vi "UHR-Fleezers Control (host) - 10.3.vi"() -> ()   [LabVIEW 2010] (continued)
        n744 = property on="Mean" class="DigNum (strict)"("Caption.Text"=w1860) -> ()  [unwired: 2 in, 2 out]
        n745 = property on="Difference" class="DigNum (strict)"("Caption.Text"=w1859) -> ()  [unwired: 2 in, 2 out]
      }
    }
    n746 = local read "Tether"() -> (w1089:bool)
    n747 = Absolute Value(x=w1062) -> (abs(x)=w1059:dbl)
    n748 = Absolute Value(x=w1061) -> (abs(x)=w1058:dbl)
    n749 = Add(x=w1059, y=w1058) -> (x+y=w1137:dbl)
    n750 = Subtract(x=w1059, y=w1058) -> (x-y=→"Difference":dbl)
    n751 = feedback #18(w1080) -> (w1079:dbl[])
    n752 = Divide(x=w1137, y=2.0) -> (x/y=w1088:dbl)
    "Mean" <- w1088
    n753 = case shown="True" w1089 {
      tunnel: w1088 -> [_ w1404]
      frame False {
      }
      frame True {
        n754 = Greater?(x="Lost Tether Alarm Threshold (pN)", y=w1404) -> (0:w1402:bool)
        n755 = case shown="True" w1402 {
          frame False {
          }
          frame True {
            n756 = flat-sequence {
              frame #0 {
                # "stop only if saving"
                n757 = local read "Saving..."() -> (w1417:bool)
                n758 = And(x=w1417, y="TA Cancel Save?") -> (x .and. y?=w1416:bool)
                n759 = local write "Stop Saving"(w1416) -> ()
              }
              frame #1 {
                n760 = case shown="True" "TA Green Off?" {
                  frame False {
                  }
                  frame True {
                    w1420 = FALSE ("Fl. Triggered...")
                    n761 = local write "Fl. Triggered..."(w1420) -> ()
                    n762 = property on="Green Laser ON/Interlacing" class="Bool (strict)"("Val(Sgnl)"=w1420) -> ()  [unwired: 2 in, 2 out]
                  }
                }
              }
            }
            n763 = local read "Time tether formed"() -> (w1411:timestamp)
            n764 = Get Date/Time In Seconds() -> (seconds since 1Jan1904=w1412:timestamp)
            n765 = Subtract(x=w1412, y=w1411) -> (x-y=w1410:dbl)
            n766 = Number To Decimal String(number=w1410) -> (decimal integer string=w1407:string)  [unwired: 1 out]
            n767 = local read "Messages"() -> (w1414:string)
            n768 = call <vilib>:"Beep.vi"() -> ()  [unwired: 3 in, 9 out]
            n769 = Concatenate Strings("Lost tether (" ("Message to add"), w1407, " s)." ("string")) -> (w1409:string)
            n770 = local write "Tether"(FALSE ("Tether")) -> ()
            n771 = call "Update messages.vi"("Message to add"=w1409, "Old message string"=w1414) -> ("New message string"=w1413:string)
            n772 = local write "Messages"(w1413) -> ()
            n773 = property on="Trap Pos. FB ON" class="Bool (strict)"("Val(Sgnl)"=FALSE ("Value (Signaling)")) -> ()  [unwired: 2 in, 2 out]
          }
        }
      }
    }
    n774 = Build Array (concatenate)(w1080, w1079) -> (w1078:dbl[])
    n775 = Split 1D Array(array=w1078, index=w957) -> (first subarray=w1074:dbl[])  [unwired: 1 out]
    n776 = feedback-in #18(w1074) -> ()
    n777 = call <vilib>:"Mean.vi"("X"=w1074) -> ("mean"=w1073:dbl)  [unwired: 1 out]
    "Bead Mean (nm)" <- w1073
    n778 = Subtract(x=w1074, y=w1073) -> (x-y=w1072:dbl[])
    n779 = Square(x=w1072) -> (x^2=w1071:dbl[])
    n780 = call <vilib>:"Mean.vi"("X"=w1071) -> ("mean"=w1070:dbl)  [unwired: 1 out]
    n781 = Square Root(x=w1070) -> (sqrt(x)=w1069:dbl)
    n782 = Multiply(x=10.0, y=w1069) -> (x*y=→"RMS (Ang)":dbl)
    n783 = xnode "Read/Write Control"("FPGA VI Reference In"=w1113, "error in"=w1112) -> ("FPGA VI Reference Out"=w1231:T19, "error out"=w1225:errorcluster, "AI2 Y Sum Set 1"=w1221:i16, "AI2 Y Sum Set 2"=w1220:i16, "AI1 X Set 1"=w992:fxp<+/-,16,1>, "AI1 X Set 2"=w991:fxp<+/-,16,1>, "Trap Pos FB Int Signal"=→"Trap Pos FB Int Signal":fxp<+/-,24,9>, "Trap Pos FB Int-Norm Signal"=→"Trap Pos FB Int-Norm Signal":fxp<+/-,16,1>, "Trap Pos FB Action"=w985:i64, "Scanning"=→"AOD Scanning":bool, "Scan I"=→"AOD Scan I":u64, "Scanning MCL"=w1223:bool, "Scan I (MCL)"=→"MCL Scan I":u64, "Green FB Signals"=w1160:T32)  [unwired: 1 out]
    "MCL Scanning" <- w1223
    "Trap Pos FB Action" <- w985
    n784 = local read "AI2 (V)"() -> (w1222:cluster{"Set 1":dbl, "Set 2":dbl})
    n785 = Bundle By Name(cluster=w1222, "Set 1"=w1221, "Set 2"=w1220) -> (w1218:cluster{"Set 1":dbl, "Set 2":dbl})
    n786 = Divide(x=w985, y=327.67) -> (x/y=→"Action (%)":dbl)
    n787 = local read "Trap X (AI1)"() -> (w1005:T10)
    n788 = Divide(x=w1218, y=3276.7) -> (x/y=w1217:cluster{"Set 1":dbl, "Set 2":dbl})
    n789 = local write "AI2 (V)"(w1217) -> ()
    n790 = Bundle(cluster=w1005, "Trap 1"=w992, "Trap 2"=w991) -> (→"Trap X (AI1)":T10)
    n791 = Divide(x=w1160, y=3276.7) -> (x/y=w1156:T41)
    n792 = Unbundle By Name(w1156) -> ("Green FB Ch 0"=w1159:dbl, "Green FB Ch 1"=w1158:dbl, "Green FB Ch 2"=w1157:dbl)
    n793 = Divide(x=w1159, y=w1157) -> (x/y=w1155:dbl)
    n794 = Divide(x=w1158, y=w1157) -> (x/y=w1154:dbl)
    n795 = flat-sequence "To save data" {
      tunnel: [w3725] -> w1243
      tunnel: [w3726] -> w1242
      tunnel: w1191 -> [w3719]
      tunnel: w1076 -> [w3723]
      tunnel: ["Save Calibration"] -> w1214
      tunnel: w1211 -> [w3722]
      tunnel: [w3715] -> w1210
      tunnel: [w3712] -> w1209
      tunnel: [w3709] -> w1208
      tunnel: w1190 -> [w3711]
      tunnel: w1095 -> [w3705]
      tunnel: [w3705] -> w1094
      tunnel: ["Start Saving"] -> w1050
      tunnel: [w3699] -> w973
      tunnel: [w3698] -> w972
      tunnel: w1243 -> [w3960]
      tunnel: w1242 -> [w3959]
      tunnel: w974 -> [w3958]
      tunnel: w1214 -> [w3957]
      tunnel: w1210 -> [w3955]
      tunnel: w1209 -> [w3954]
      tunnel: w1208 -> [w3953]
      tunnel: w1063 -> [w3952]
      tunnel: w1105 -> [w3951]
      tunnel: w1094 -> [w3950]
      tunnel: w1050 -> [w3949]
      tunnel: w1048 -> [w3948]
      tunnel: w1024 -> [w3947]
      tunnel: w973 -> [w3946]
      tunnel: w972 -> [w3945]
      tunnel: w971 -> [w3944]
      frame #0 {
        n796 = Or(x="Save N Sets", y="Start Saving") -> (x .or. y?=w3706:bool)
        n797 = To Double Precision Float(number=w3722) -> (double precision float=w3716:dbl)
        n798 = Build Array(w3706, "Save Calibration", w3719, w3711) -> (w3721:bool[])
        n799 = Compound Arithmetic op=OR("Save Calibration", w3719, w3706, w3711) -> (w3724:bool)
        n800 = Boolean Array To Number(Boolean array=w3721) -> (number=w3718:u32)
        n801 = feedback #19(FALSE ("Save APD Data\nwith Trap Data")) -> (w3700:bool)
        n802 = feedback #20(refnum<k0> refnum) -> (w3727:refnum<file>)
        n803 = feedback #21(refnum<k0> refnum) -> (w3702:refnum<file>)
        n804 = feedback #22(FALSE ("Save APD Data\nwith Trap Data")) -> (w3710:bool)
        n805 = feedback #23(refnum<k0> refnum) -> (w3713:refnum<file>)
        n806 = feedback #24(0) -> (w3729:i32)
        n807 = feedback #25() -> (w3717:u32)  [unwired: 1 out]
        n808 = case shown="True" w3724 {
          tunnel: [w3736 1] -> w3725
          tunnel: w3729 -> [w3738 _]
          tunnel: [w3737 w3756] -> w3726
          tunnel: w3727 -> [w3737 _]
          tunnel: w3723 -> [_ w3776]
          tunnel: w3716 -> [_ w3774]
          tunnel: w3718 -> [_ w3777]
          tunnel: [w3735 w3755] -> w3715
          tunnel: w3717 -> [w3735 _]
          tunnel: [w3734 w3753] -> w3712
          tunnel: w3713 -> [w3734 _]
          tunnel: [w3733 w3752] -> w3709
          tunnel: w3710 -> [w3733 _]
          tunnel: "Start Saving" -> [_ w3750]
          tunnel: w3705 -> [_ w3749]
          tunnel: [w3732 w3740] -> w3698
          tunnel: w3702 -> [w3732 _]
          tunnel: [w3731 w3739] -> w3699
          tunnel: w3700 -> [w3731 _]
          frame False {
            n809 = Increment(x=w3738) -> (x+1=w3736:i32)
          }
          frame True {
            w3746 = FALSE ("Start Saving")
            w3751 = 9.0  # File Version
            w3759 = FALSE ("prepend array or string size? (T)")
            w3757 = T34."big-endian, network order" ("byte order (0:big-endian, network order)")
            n810 = local read "BD 1 Frequency 1 (MHz)"() -> (w3773:dbl)
            n811 = local read "BD 2 Frequency 1 (MHz)"() -> (w3772:dbl)
            n812 = local read "BD 1 Frequency 2 (MHz)"() -> (w3771:dbl)
            n813 = local read "BD 2 Frequency 2 (MHz)"() -> (w3770:dbl)
            n814 = local read "BD 1 Frequency 3 (MHz)"() -> (w3769:dbl)
            n815 = local read "BD 2 Frequency 3 (MHz)"() -> (w3768:dbl)
            n816 = Array Size(array=w3749) -> (size(s)=w3748:i32)
            n817 = To Double Precision Float(number=w3748) -> (double precision float=w3747:dbl)
            n818 = local write "Save Calibration"(w3746) -> ()
            n819 = local write "Start Saving"(w3746) -> ()
            n820 = Build Array("Save APD Data\nwith Trap Data", "Save Trap Pos. Data") -> (w3743:bool[])
            n821 = Boolean Array To Number(Boolean array=w3743) -> (number=w3742:u32)
            n822 = Build Array(w3773, w3772, w3771, w3770, w3769, w3768) -> (w3767:dbl[])
            n823 = case shown="4" w3777 {
              tunnel: w3776 -> [w3848 w3868 w3884 w3922]
              tunnel: w3747 -> [w3853 w3875 w3904 w3941]
              tunnel: w3774 -> [w3852 w3874 w3903 w3940]
              tunnel: [w3849 w3870 w3895 w3932] -> w3765
              tunnel: [w3840 "Cal sets to save" w3885 w3923] -> w3755
              tunnel: w3767 -> [w3850 w3871 w3897 w3934]
              tunnel: "Save APD Data\nwith Trap Data" -> [w3847 _ w3881 w3920]
              tunnel: [w3847 w3862 w3881 w3920] -> w3752
              tunnel: w3751 -> [w3843 w3863 w3879 w3918]
              tunnel: w3750 -> [w3842 _ _ _]
              tunnel: [w3833 w3862 w3878 w3908] -> w3739
              tunnel: "Save Trap Pos. Data" -> [w3833 _ w3878 w3908]
              tunnel: w3742 -> [w3832 _ w3877 w3907]
              frame 1, Default {
                # "timeseries"
                n824 = case shown="True" "Profile" {
                  tunnel: [w3856 w3860] -> w3837
                  tunnel: [w3856 w3859] -> w3836
                  tunnel: [w3856 w3858] -> w3835
                  tunnel: [w3856 w3857] -> w3834
                  frame False {
                    w3856 = 0.0 ("f")
                  }
                  frame True {
                    n825 = local read "Current Position"() -> (w3861:cluster{dbl, dbl, dbl})
                    n826 = local read "Y change (mm)"() -> (w3857:dbl)
                    n827 = Unbundle(w3861) -> (w3860:dbl, w3859:dbl, w3858:dbl)
                  }
                }
                n828 = local read "Save ave N"() -> (w3855:dbl)
                n829 = Multiply(x=w3855, y=w3848) -> (x*y=w3854:dbl)
                n830 = To Double Precision Float(number=w3832) -> (double precision float=w3846:dbl)
                n831 = Build Array(w3843, w3848, w3854, w3853, w3852, 0.0 ("f")) -> (w3851:dbl[])
                n832 = Build Array(w3846, w3837, w3836, w3835, w3834) -> (w3844:dbl[])
                n833 = Select(t=u32 4000000000, s=w3842, f="N sets to save") -> (s? t:f=w3840:u32)
                n834 = Build Array (concatenate)(w3851, w3850, w3844) -> (w3849:dbl[])
              }
              frame 2 {
                w3865 = 0.0 ("f")
                w3862 = FALSE ("Save APD Data\nwith Trap Data")
                # "calibration"
                n835 = Boolean To (0,1)(Boolean=w3862) -> (0, 1=w3867:i16)
                n836 = To Double Precision Float(number=w3867) -> (double precision float=w3866:dbl)
                n837 = Build Array(w3866, w3865, w3865, w3865, w3865) -> (w3864:dbl[])
                n838 = Build Array(w3863, w3868, w3868, w3875, w3874, 1.0 ("t")) -> (w3872:dbl[])
                n839 = Build Array (concatenate)(w3872, w3871, w3864) -> (w3870:dbl[])
                "Calibrating Trap..." <- TRUE ("Calibrating...")
              }
              frame 4 {
                w3882 = 0.0 ("f")
                # "scan dir (x/y = 0/1)"
                # "cycles/step"
                # "n scans (f/b)"
                # "steps"
                # "freq. range"
                # "AOD raster scan"
                n840 = local read "Number of F/B Scans (AOD)"() -> (w3889:u16)
                n841 = local read "Cycles/step (AOD)"() -> (w3891:u64)
                n842 = local read "Scan Range (MHz)"() -> (w3894:dbl)
                n843 = local read "Scan steps (AOD)"() -> (w3893:u64)
                n844 = local read "Scan BD"() -> (w3901:bool)
                n845 = local read "Save ave N"() -> (w3906:dbl)
                n846 = Boolean To (0,1)(Boolean=w3901) -> (0, 1=w3900:i16)
                n847 = To Double Precision Float(number=w3889) -> (double precision float=w3888:dbl)
                n848 = To Double Precision Float(number=w3893) -> (double precision float=w3892:dbl)
                n849 = To Double Precision Float(number=w3891) -> (double precision float=w3890:dbl)
                n850 = To Double Precision Float(number=w3900) -> (double precision float=w3899:dbl)
                n851 = Multiply(x=w3906, y=w3884) -> (x*y=w3905:dbl)
                n852 = To Double Precision Float(number=w3877) -> (double precision float=w3883:dbl)
                n853 = Build Array(w3883, w3882, w3882, w3882, w3882) -> (w3880:dbl[])
                n854 = local read "N sets should be saved"() -> (w3886:dbl)
                n855 = Build Array(w3899, w3894, w3892, w3890, w3888) -> (w3896:dbl[])
                n856 = Build Array(w3879, w3884, w3905, w3904, w3903, 2.0 ("t")) -> (w3898:dbl[])
                n857 = Round Toward +Infinity(x=w3886) -> (ceil(x): smallest int >= x=w3887:dbl)
                n858 = Build Array (concatenate)(w3898, w3897, w3880, w3896) -> (w3895:dbl[])
                n859 = To Unsigned Long Integer(number=w3887) -> (unsigned 32bit integer=w3885:u32)
              }
              frame 8 {
                w3915 = 0.0 ("f")
                # "MCL raster scan"
                n860 = local read "Number of scans (MCL)"() -> (w3910:u64)
                n861 = local read "Scan lines (y)"() -> (w3909:u64)
                n862 = local read "2D or 1D Scan"() -> (w3912:bool)
                n863 = local read "Scan Range (V)\n(of steps)"() -> (w3931:dbl)
                n864 = local read "Fast Scan Dir"() -> (w3938:bool)
                n865 = local read "Cycles/step (MCL)"() -> (w3928:u64)
                n866 = local read "Scan steps (MCL)"() -> (w3930:u64)
                n867 = Select(t=w3909, s=w3912, f=w3910) -> (s? t:f=w3911:u64)
                n868 = Boolean To (0,1)(Boolean=w3912) -> (0, 1=w3914:i16)
                n869 = local read "Save ave N"() -> (w3943:dbl)
                n870 = local read "Initial X"() -> (w3917:dbl)
                n871 = local read "Initial Y"() -> (w3916:dbl)
                n872 = To Double Precision Float(number=w3914) -> (double precision float=w3913:dbl)
                n873 = Boolean To (0,1)(Boolean=w3938) -> (0, 1=w3937:i16)
                n874 = To Double Precision Float(number=w3911) -> (double precision float=w3926:dbl)
                n875 = To Double Precision Float(number=w3930) -> (double precision float=w3929:dbl)
                n876 = To Double Precision Float(number=w3928) -> (double precision float=w3927:dbl)
                n877 = To Double Precision Float(number=w3937) -> (double precision float=w3936:dbl)
                n878 = Multiply(x=w3943, y=w3922) -> (x*y=w3942:dbl)
                n879 = To Double Precision Float(number=w3907) -> (double precision float=w3921:dbl)
                n880 = local read "N sets should be saved (MCL)"() -> (w3924:dbl)
                n881 = Build Array(w3921, w3913, w3915, w3915, w3915) -> (w3919:dbl[])
                n882 = Build Array(w3936, w3931, w3929, w3927, w3926, w3917, w3916) -> (w3933:dbl[])
                n883 = Build Array(w3918, w3922, w3942, w3941, w3940, 3.0 ("t")) -> (w3935:dbl[])
                n884 = Round Toward +Infinity(x=w3924) -> (ceil(x): smallest int >= x=w3925:dbl)
                n885 = Build Array (concatenate)(w3935, w3934, w3919, w3933) -> (w3932:dbl[])
                n886 = To Unsigned Long Integer(number=w3925) -> (unsigned 32bit integer=w3923:u32)
              }
            }
            n887 = local read "Index"() -> (w3782:dbl)
            n888 = call "Create new save file.vi"("Insert"="", "Ext"=".dat", "Index In"=w3782) -> ("Path Out"=w3741:path, "Index Out"=w3754:dbl)
            n889 = local write "Save file name"(w3741) -> ()
            n890 = local write "Index"(w3754) -> ()
            n891 = local write "Save index"(w3754) -> ()
            n892 = Array Size(array=w3765) -> (size(s)=w3766:i32)
            n893 = Open/Create/Replace File(file path (use dialog)=w3741, operation (0:open)=T33."create", access (0:read/write)=enum16{"read/write", "read-only", "write-only"}."write-only") -> (refnum out=w3779:refnum<file>)  [unwired: 1 in, 4 out]
            n894 = local write "Saving..."(TRUE ("Saving...")) -> ()
            n895 = To Double Precision Float(number=w3766) -> (double precision float=w3764:dbl)
            n896 = String Length(string="Comment (data description)") -> (length=w3762:i32)
            n897 = To Double Precision Float(number=w3762) -> (double precision float=w3761:dbl)
            n898 = Deny Access(7:w3779) -> (3:w3778:refnum<file>)  [unwired: 1 in, 2 out]
            n899 = Build Array (concatenate)(w3764, w3765, w3761) -> (w3763:dbl[])
            n900 = case "If fluorescence data to be saved" shown="True" w3752 {
              tunnel: w3741 -> [_ w3831]
              tunnel: [refnum<k0> refnum w3811] -> w3753
              frame False {
              }
              frame True {
                w3810 = 0.0
                n901 = local read "APD Integration Time (s)"() -> (w3816:dbl)
                n902 = local read "N APD Samp/step"() -> (w3809:dbl)
                n903 = Path To String(path=w3831) -> (string=w3830:string)
                n904 = String Length(string=w3830) -> (length=w3829:i32)
                n905 = Subtract(x=w3829, y=4) -> (x-y=w3827:i32)
                n906 = String Subset(string=w3830, length (rest)=w3827) -> (substring=w3826:string)  [unwired: 1 out]
                n907 = Build Array(w3816, w3809, w3810, w3810, w3810, w3810, w3810, w3810) -> (w3813:dbl[])
                n908 = Concatenate Strings(w3826, "_fl.dat" ("string")) -> (w3824:string)
                n909 = Array Size(array=w3813) -> (size(s)=w3815:i32)
                n910 = String To Path(string=w3824) -> (path=w3820:path)
                n911 = Open/Create/Replace File(file path (use dialog)=w3820, operation (0:open)=T33."create", access (0:read/write)=enum16{"read/write", "read-only", "write-only"}."write-only") -> (refnum out=w3821:refnum<file>)  [unwired: 1 in, 4 out]
                n912 = Deny Access(7:w3821) -> (3:w3817:refnum<file>)  [unwired: 1 in, 2 out]
                n913 = To Double Precision Float(number=w3815) -> (double precision float=w3814:dbl)
                n914 = Build Array (concatenate)(w3814, w3813) -> (w3812:dbl[])
                n915 = Write to Binary File(file (use dialog)=w3817, data=w3812, 5:FALSE ("prepend array or string size? (T)"), 9:T34."big-endian, network order" ("byte order (0:big-endian, network order)")) -> (refnum out=w3811:refnum<file>)  [unwired: 1 in, 3 out]
              }
            }
            n916 = case shown="True" w3739 {
              tunnel: w3741 -> [_ w3793]
              tunnel: [refnum<k0> refnum w3792] -> w3740
              frame False {
              }
              frame True {
                w3788 = 0.0 ("element")
                n917 = Path To String(path=w3793) -> (string=w3807:string)
                n918 = Build Array(w3788, w3788, w3788, w3788, w3788, w3788, w3788, w3788) -> (w3789:dbl[])
                n919 = String Length(string=w3807) -> (length=w3806:i32)
                n920 = Subtract(x=w3806, y=4) -> (x-y=w3804:i32)
                n921 = Array Size(array=w3789) -> (size(s)=w3791:i32)
                n922 = String Subset(string=w3807, length (rest)=w3804) -> (substring=w3803:string)  [unwired: 1 out]
                n923 = To Double Precision Float(number=w3791) -> (double precision float=w3790:dbl)
                n924 = Concatenate Strings(w3803, "_pos.dat" ("string")) -> (w3801:string)
                n925 = Build Array (concatenate)(w3790, w3789) -> (w3787:dbl[])
                n926 = String To Path(string=w3801) -> (path=w3797:path)
                n927 = Open/Create/Replace File(file path (use dialog)=w3797, operation (0:open)=T33."create", access (0:read/write)=enum16{"read/write", "read-only", "write-only"}."write-only") -> (refnum out=w3798:refnum<file>)  [unwired: 1 in, 4 out]
                n928 = Deny Access(7:w3798) -> (3:w3794:refnum<file>)  [unwired: 1 in, 2 out]
                n929 = Write to Binary File(file (use dialog)=w3794, data=w3787, 5:FALSE ("prepend array or string size? (T)"), 9:T34."big-endian, network order" ("byte order (0:big-endian, network order)")) -> (refnum out=w3792:refnum<file>)  [unwired: 1 in, 3 out]
              }
            }
            n930 = Write to Binary File(file (use dialog)=w3778, data=w3763, 5:w3759, 9:w3757) -> (refnum out=w3760:refnum<file>)  [unwired: 1 in, 3 out]
            n931 = Write to Binary File(file (use dialog)=w3760, data="Comment (data description)", 5:w3759, 9:w3757) -> (refnum out=w3756:refnum<file>)  [unwired: 1 in, 3 out]
          }
        }
        n932 = feedback-in #19(w3699) -> ()
        n933 = feedback-in #20(w3726) -> ()
        n934 = feedback-in #21(w3698) -> ()
        n935 = feedback-in #22(w3709) -> ()
        n936 = feedback-in #23(w3712) -> ()
        n937 = feedback-in #24(w3725) -> ()
        n938 = feedback-in #25(w3715) -> ()
      }
      frame #1 {
        n939 = local read "Saving..."() -> (w3956:bool)
        n940 = case shown="True" w3956 {
          tunnel: w3960 -> [_ w3970]
          tunnel: w3959 -> [_ w3984]
          tunnel: w3958 -> [_ w3980]
          tunnel: w3957 -> [_ w3979]
          tunnel: w3955 -> [_ w3978]
          tunnel: w3954 -> [_ w3973]
          tunnel: w3953 -> [_ w3972]
          tunnel: w3952 -> [_ w3971]
          tunnel: w3951 -> [_ w3969]
          tunnel: w3950 -> [_ w3967]
          tunnel: w3949 -> [_ w3966]
          tunnel: w3948 -> [_ w3965]
          tunnel: w3947 -> [_ w3964]
          tunnel: w3946 -> [_ w3963]
          tunnel: w3945 -> [_ w3962]
          tunnel: w3944 -> [_ w3961]
          frame False {
          }
          frame True {
            n941 = Multiply(x=w3970, y=w3969) -> (x*y=→"Time (s)":dbl)
            n942 = Less Or Equal?(x=w3970, y=w3978) -> (x <= y?=w3982:bool)
            n943 = Or(x="Stop Saving", y="Abort save 2") -> (x .or. y?=w3974:bool)
            n944 = Not(x=w3974) -> (.not. x?=w3983:bool)
            n945 = And(x=w3982, y=w3983) -> (x .and. y?=w3981:bool)
            n946 = case shown="True" w3981 {
              tunnel: w3984 -> [w3991 w4059]
              tunnel: [0.0 w4062] -> w3977
              tunnel: w3970 -> [_ w4060]
              tunnel: w3978 -> [_ w4061]
              tunnel: w3980 -> [_ w4056]
              tunnel: w3979 -> [_ _]
              tunnel: w3973 -> [w3989 w4049]
              tunnel: w3972 -> [w3988 w4050]
              tunnel: w3971 -> [_ w4048]
              tunnel: w3967 -> [_ w4047]
              tunnel: w3966 -> [_ w4001]
              tunnel: w3965 -> [_ w4040]
              tunnel: w3964 -> [_ w4018]
              tunnel: w3963 -> [w3985 w3999]
              tunnel: w3962 -> [w3986 w3998]
              tunnel: w3961 -> [_ w3995]
              frame False {
                w3987 = FALSE
                n947 = Close File(refnum=w3991) -> ()  [unwired: 1 in, 2 out]
                n948 = case shown="True" w3988 {
                  tunnel: w3989 -> [_ w3993]
                  frame False {
                  }
                  frame True {
                    n949 = Close File(refnum=w3993) -> ()  [unwired: 1 in, 2 out]
                  }
                }
                n950 = case shown="True" w3985 {
                  tunnel: w3986 -> [_ w3992]
                  frame False {
                  }
                  frame True {
                    n951 = Close File(refnum=w3992) -> ()  [unwired: 1 in, 2 out]
                  }
                }
                n952 = local write "Raster Scanning..."(w3987) -> ()
                n953 = local write "Calibrating Trap..."(w3987) -> ()
                n954 = call <vilib>:"Beep.vi"() -> ()  [unwired: 3 in, 9 out]
                n955 = local write "Stop Saving"(w3987) -> ()
                "Saving..." <- w3987
              }
              frame True {
                n956 = local read "Calibrating Trap..."() -> (w4051:bool)
                n957 = case "Write fl. data" shown="True" w4050 {
                  tunnel: w4049 -> [_ w4085]
                  tunnel: w4048 -> [_ w4084]
                  frame False {
                  }
                  frame True {
                    n958 = Write to Binary File(file (use dialog)=w4085, data=w4084, 5:FALSE ("prepend array or string size? (T)"), 9:T34."big-endian, network order" ("byte order (0:big-endian, network order)")) -> ()  [unwired: 1 in, 4 out]
                  }
                }
                n959 = Greater?(x="Save ave N", y=1.0) -> (0:w4054:bool)
                n960 = Not(x=w4051) -> (.not. x?=w4053:bool)
                n961 = And(x=w4053, y=w4054) -> (x .and. y?=w3996:bool)
                n962 = case shown="True" w3996 {
                  tunnel: w3995 -> [w4065 w4076]
                  tunnel: [w4065 w4068] -> w3994
                  tunnel: "Save ave N" -> [_ w4069]
                  frame False {
                  }
                  frame True {
                    w4066 = 2 ("dimension size")
                    n963 = Array Size(array=w4076) -> (size(s)=w4070:i32)
                    n964 = Divide(x=w4070, y=w4066) -> (x/y=w4074:dbl)
                    n965 = Reshape Array(w4076, w4074, w4066) -> (w4075:u64[][])
                    n966 = Transpose 2D Array(2D array=w4075) -> (transposed array=w4073:u64[][])
                    n967 = for {
                      tunnel: w4073 -> [w4078] mode=indexing
                      tunnel: [w4077] -> w4067 mode=indexing
                      tunnel: w4069 -> [w4079]
                      workers-P: _ -> [_]
                      n968 = call "downsample 1D array - U64.vi"("Ave N"=w4079, "Array In"=w4078) -> ("Array Out"=w4077:u64[])  [unwired: 1 in]
                    }
                    n969 = Transpose 2D Array(2D array=w4067) -> (transposed array=w4072:u64[][])
                    n970 = Divide(x=w4070, y=w4069) -> (x/y=w4071:dbl)
                    n971 = Reshape Array(w4072, w4071) -> (w4068:u64[])
                  }
                }
                n972 = case shown="True" w3996 {
                  tunnel: w4056 -> [w4088 w4100]
                  tunnel: [w4088 w4092] -> w4052
                  tunnel: "Save ave N" -> [_ w4093]
                  tunnel: w4047 -> [_ w4091]
                  frame False {
                  }
                  frame True {
                    n973 = Array Size(array=w4100) -> (size(s)=w4094:i32)
                    n974 = Array Size(array=w4091) -> (size(s)=w4090:i32)
                    n975 = Divide(x=w4094, y=w4090) -> (x/y=w4098:dbl)
                    n976 = Reshape Array(w4100, w4098, w4090) -> (w4099:i16[][])
                    n977 = Transpose 2D Array(2D array=w4099) -> (transposed array=w4097:i16[][])
                    n978 = for {
                      tunnel: w4097 -> [w4103] mode=indexing
                      tunnel: [w4102] -> w4089 mode=indexing
                      tunnel: w4093 -> [w4101]
                      workers-P: _ -> [_]
                      n979 = call "downsample 1D array - I16.vi"("Ave N"=w4101, "Array In"=w4103) -> ("Array Out"=w4102:i16[])  [unwired: 1 out]
                    }
                    n980 = Transpose 2D Array(2D array=w4089) -> (transposed array=w4096:i16[][])
                    n981 = Divide(x=w4094, y=w4093) -> (x/y=w4095:dbl)
                    n982 = Reshape Array(w4096, w4095) -> (w4092:i16[])
                  }
                }
                n983 = Index Array(array=w4018, index=1) -> (element=w4021:waveform(dbl))
                n984 = Index Array(array=w4018, index=0) -> (element=w4023:waveform(dbl))
                n985 = Unbundle By Name(w4021) -> ("Y"=w4025:dbl[])
                n986 = Unbundle By Name(w4023) -> ("Y"=w4033:dbl[])
                n987 = case "Write trap pos. data" shown="True" w3999 {
                  tunnel: w3998 -> [_ w4081]
                  tunnel: w3994 -> [_ w4080]
                  frame False {
                  }
                  frame True {
                    n988 = Write to Binary File(file (use dialog)=w4081, data=w4080, 5:FALSE ("prepend array or string size? (T)"), 9:T34."big-endian, network order" ("byte order (0:big-endian, network order)")) -> ()  [unwired: 1 in, 4 out]
                  }
                }
                n989 = Write to Binary File(file (use dialog)=w4059, data=w4052, 5:FALSE ("prepend array or string size? (T)"), 9:T34."big-endian, network order" ("byte order (0:big-endian, network order)")) -> ()  [unwired: 1 in, 4 out]
                n990 = feedback #26(w4025) -> (w4027:dbl[])
                n991 = Build Array (concatenate)(w4027, w4025) -> (w4026:dbl[])
                n992 = Select(t=w4025, s=w4001, f=w4026) -> (s? t:f=w4011:dbl[])
                n993 = feedback-in #26(w4011) -> ()
                n994 = feedback #27(w4033) -> (w4046:dbl[])
                n995 = Build Array (concatenate)(w4046, w4033) -> (w4045:dbl[])
                n996 = Select(t=w4033, s=w4001, f=w4045) -> (s? t:f=w4020:dbl[])
                n997 = feedback-in #27(w4020) -> ()
                n998 = Divide(x=w4060, y=w4061) -> (x/y=w4063:dbl)
                n999 = Multiply(x=w4063, y=100.0) -> (x*y=w4062:dbl)
                n1000 = Build Array(w4020, w4011) -> (→"Saved APD":dbl[][])
                n1001 = Array Size(array=w4020) -> (size(s)=w4038:i32)
                n1002 = Unbundle By Name(w4040) -> ("Y"=w4044:dbl[])
                n1003 = Subtract(x=w4038, y="N pts to average") -> (x-y=w4014:i32)
                n1004 = Multiply(x="N pts to average", y=u16 2) -> (x*y=w4015:u16)
                n1005 = Subtract(x=w4038, y=w4015) -> (x-y=w4013:i32)
                n1006 = feedback #28(w4044) -> (w4043:dbl[])
                n1007 = Build Array (concatenate)(w4043, w4044) -> (w4042:dbl[])
                n1008 = Select(t=w4044, s=w4001, f=w4042) -> (s? t:f=w4041:dbl[])
                "Trap Delta Graph" <- w4041
                n1009 = feedback-in #28(w4041) -> ()
                n1010 = Array Subset(array=w4020, index=w4014, length="N pts to average") -> (w4037:dbl[])
                n1011 = Array Subset(array=w4020, index=w4013, length="N pts to average") -> (w4036:dbl[])
                n1012 = Array Subset(array=w4011, index=w4014, length="N pts to average") -> (w4017:dbl[])
                n1013 = Array Subset(array=w4011, index=w4013, length="N pts to average") -> (w4016:dbl[])
                n1014 = call <vilib>:"Mean.vi"("X"=w4037) -> ("mean"=w4035:dbl)  [unwired: 1 out]
                n1015 = call <vilib>:"Mean.vi"("X"=w4017) -> ("mean"=w4010:dbl)  [unwired: 1 out]
                n1016 = call <vilib>:"Mean.vi"("X"=w4036) -> ("mean"=w4034:dbl)  [unwired: 1 out]
                n1017 = call <vilib>:"Mean.vi"("X"=w4016) -> ("mean"=w4009:dbl)  [unwired: 1 out]
                n1018 = Subtract(x=w4010, y=w4009) -> (x-y=w4000:dbl)
                "Delta Fl. 2" <- w4000
                n1019 = Subtract(x=w4035, y=w4034) -> (x-y=w4032:dbl)
                "Delta Fl. 1" <- w4032
                n1020 = Initialize Array(w4032, 1 ("dimension size")) -> (w4029:dbl[])
                n1021 = Initialize Array(w4000, 1 ("dimension size")) -> (w4006:dbl[])
                n1022 = feedback #29(w4029) -> (w4030:dbl[])
                n1023 = Build Array (concatenate)(w4030, w4029) -> (w4028:dbl[])
                n1024 = feedback #30(w4006) -> (w4007:dbl[])
                n1025 = Build Array (concatenate)(w4007, w4006) -> (w4005:dbl[])
                n1026 = Select(t=w4029, s=w4001, f=w4028) -> (s? t:f=w4004:dbl[])
                n1027 = feedback-in #29(w4004) -> ()
                n1028 = Select(t=w4006, s=w4001, f=w4005) -> (s? t:f=w4003:dbl[])
                n1029 = feedback-in #30(w4003) -> ()
                n1030 = Build Array(w4004, w4003) -> (→"Save APD Deriv":dbl[][])
              }
            }
            "Progress" <- w3977
            "Progress 2" <- w3977
          }
        }
      }
    }
    n1031 = Bundle By Name(cluster=w1156, "Green FB Ch 0"=w1155, "Green FB Ch 1"=w1154) -> (w1134:T41)
    "Green FB Signals (V)" <- w1134
    n1032 = Unbundle By Name(w1134) -> ("Green FB Ch 2"=→"Green FB Plot":dbl)
    n1033 = local read "wait to reset values"() -> (w1226:bool)
    n1034 = Not(x=w1223) -> (.not. x?=w1227:bool)
    n1035 = And(x=w1227, y=w1226) -> (x .and. y?=w1228:bool)
    n1036 = case "Part of MCL raster scanning: returns to initial positions after scan done" shown="True" w1228 {
      tunnel: w1231 -> [w2625 w2632]
      tunnel: [w2625 w2631] -> w1230
      tunnel: w1225 -> [w2624 w2630]
      tunnel: [w2624 w2629] -> w1224
      frame False {
      }
      frame True {
        w2640 = 10.0 ("y")
        w2639 = 32767.0 ("y")
        # "to return scan values\nafter a synchronous \nAOM scan"
        n1037 = local read "AO2"() -> (w2633:dbl)
        n1038 = local read "AO1"() -> (w2634:dbl)
        n1039 = local write "wait to reset values"(FALSE ("wait to reset values")) -> ()
        n1040 = Multiply(x=w2634, y=w2639) -> (x*y=w2636:dbl)
        n1041 = Multiply(x=w2633, y=w2639) -> (x*y=w2638:dbl)
        n1042 = Divide(x=w2636, y=w2640) -> (x/y=w2635:dbl)
        n1043 = Divide(x=w2638, y=w2640) -> (x/y=w2637:dbl)
        n1044 = To Word Integer(number=w2635) -> (16bit integer=w2641:i16)
        n1045 = To Word Integer(number=w2637) -> (16bit integer=w2642:i16)
        n1046 = local read "Total Counts (ticks)"() -> (w2626:u32)
        n1047 = xnode "Read/Write Control"("FPGA VI Reference In"=w2632, "error in"=w2630, "AO1"=w2641, "AO2"=w2642, "MCL count"=w2626) -> ("FPGA VI Reference Out"=w2631:T19, "error out"=w2629:errorcluster)
        n1048 = local read "Scan Range (V)\n(of steps)"() -> (w2627:dbl)
        n1049 = property on="Scan Range (V)\n(of steps)" class="DigNum (strict)"("Val(Sgnl)"=w2627) -> ()  [unwired: 2 in, 2 out]
      }
    }
    n1050 = node-c288() -> ()  [unwired: 2 out]
  }
  n1051 = timed-loop "Control parameters (event loop)" {
    tunnel: w8 -> [w4180]
    shift-right: [w4179] -> _
    shift-left: errorcluster {"status"=FALSE, "code"=0, "source"=""} ("error out") -> [w4178]
    tunnel: [w4177] -> w202
    timing: w49 -> [_]
    timing-out: [_] -> w48
    tunnel: w22 -> [w4176]
    stop <- w4177 stop-if-true
    n1052 = node-c288() -> ()  [unwired: 2 out]
    n1053 = event shown="[30] \"Freq or Amp switch first\", \"Swap F1 and F2\", \"Freq switch delay\", \"Amp switch delay\": Value Change" {
      selector: _ -> [_ _ _ _ _ _ _ _ _ _ _ _ _ _ _ _ _ _ _ _ _ _ _ _ _ _ _ _ _ _ _ _ _ _ _ _ _ _ _ _ _ _ _ _ _ _ _ _ _ _ _ _ _]
      dyn-events: _ -> [_ _ _ _ _ _ _ _ _ _ _ _ _ _ _ _ _ _ _ _ _ _ _ _ _ _ _ _ _ _ _ _ _ _ _ _ _ _ _ _ _ _ _ _ _ _ _ _ _ _ _ _ _]
      timeout: _ -> [_ _ _ _ _ _ _ _ _ _ _ _ _ _ _ _ _ _ _ _ _ _ _ _ _ _ _ _ _ _ _ _ _ _ _ _ _ _ _ _ _ _ _ _ _ _ _ _ _ _ _ _ _]
      tunnel: w4180 -> [w4218 _ _ _ w4340 _ w4437 _ _ _ _ w4503 _ _ w4605 w4749 w4813 w4888 w5042 w5119 w5250 w5346 w5432 w5518 w5604 w5690 w5776 w5869 w6033 w6244 w6387 w6524 _ w6731 w6773 w6821 w6900 w6942 _ w6988 _ _ _ _ w7171 _ w7264 w7305 w7352 w7540 w7589 _ w7651]
      tunnel: [w4217 _ _ _ w4330 _ w4436 _ _ w4468 _ w4482 _ _ w4604 w4745 w4810 w4885 w5041 w5117 w5249 w5340 w5426 w5512 w5598 w5684 w5770 w5867 w6032 w6242 w6385 w6522 _ w6729 w6771 w6811 w6898 w6940 _ w6986 _ _ _ _ w7169 _ _ _ _ _ _ _ _] -> w4179
      tunnel: w4178 -> [w4216 _ _ _ w4339 _ w4435 _ _ w4468 _ w4502 _ _ w4603 w4744 w4809 w4884 w5040 w5118 w5248 w5345 w5431 w5517 w5603 w5689 w5775 w5868 w6031 w6243 w6386 w6523 _ w6730 w6772 w6820 w6899 w6941 _ w6987 _ _ _ _ w7170 _ w7263 w7304 w7351 w7539 w7588 _ w7650]
      tunnel: [_ _ _ _ _ _ _ _ _ w4467 _ _ _ _ _ _ _ _ _ _ _ _ _ _ _ _ _ _ _ _ _ _ _ _ _ _ _ _ _ _ _ _ _ _ _ _ _ _ _ _ _ _ _] -> w4177
      tunnel: [_ _ _ _ _ _ _ "Round T1 X" _ _ _ _ _ _ _ _ _ _ _ _ _ _ _ _ _ _ _ _ _ _ _ _ _ _ _ _ _ _ _ _ _ _ _ _ _ _ _ _ _ _ _ _ _] -> _
      tunnel: [_ _ _ "Adjust Scale\nto Mean" _ _ _ _ _ _ _ _ _ _ _ _ _ _ _ _ _ _ _ _ _ _ _ _ _ _ _ _ _ _ _ _ _ _ _ _ _ _ _ _ _ _ _ _ _ _ "Set SP to Reading" _ _] -> _
      tunnel: [_ _ _ _ _ _ _ _ "Round T2 X" _ "Delayed Interlace Start" _ _ _ _ _ _ _ _ _ _ _ _ _ _ _ _ _ _ _ _ _ _ _ _ _ _ _ _ _ _ _ _ _ _ _ _ _ _ _ _ _ _] -> _
      tunnel: w4176 -> [_ _ _ _ _ _ _ _ _ _ _ _ _ _ _ _ _ _ _ _ _ _ _ _ _ _ _ _ _ _ _ _ _ _ _ _ _ _ _ _ _ _ _ w7162 _ _ _ _ _ _ _ _ _]
      event "AI Count (ticks)", "Sets to FIFO (Traps)", "Save ave N", "FPGA Ave.", "# Samples/channel", "N sets to save": Value Change {
        # "So that if 'Save ave N' is updated, the AOD scanning code updates too."
        n1054 = event-data() -> ()  [unwired: 6 out]
        n1055 = local read "AI Count (ticks)"() -> (w4198:u32)
        n1056 = Boolean To (0,1)(Boolean="Sets to FIFO (Traps)") -> (0, 1=w4208:cluster{"Set 1":i16, "Set 2":i16, "Set 3":i16})
        n1057 = xnode "Read/Write Control"("FPGA VI Reference In"=w4218, "error in"=w4216, "ai count"=w4198, "AI1 Sets to FIFO"="Sets to FIFO (Traps)", "N of AI1 Int Acq Sets"="N Acq Sets (Traps + Fl.)") -> ("error out"=w4217:errorcluster)  [unwired: 1 out]
        n1058 = Cluster To Array(cluster=w4208) -> (array=w4207:i16[])
        n1059 = To Unsigned Long Integer(number=w4207) -> (unsigned 32bit integer=w4187:u32[])
        n1060 = local read "Scan steps (AOD)"() -> (w4209:u64)
        n1061 = Multiply(x=w4198, y="N Acq Sets (Traps + Fl.)") -> (x*y=w4196:u32)
        n1062 = Divide(x=40000000.0, y=w4198) -> (x/y=w4190:dbl)
        "AI rate (Hz)" <- w4190
        "Ave. Rate (Hz)" <- w4190
        n1063 = Add Array Elements(numeric array=w4187) -> (sum=w4199:u32)
        "Trap Sets" <- w4199
        n1064 = Reciprocal(x=w4190) -> (1/x=→"Ave. Period (s)":dbl)
        n1065 = property on="Scan steps (AOD)" class="DigNum (strict)"("Val(Sgnl)"=w4209) -> ()  [unwired: 2 in, 2 out]
        n1066 = Divide(x=w4190, y="N Acq Sets (Traps + Fl.)") -> (x/y=w4213:dbl)
        "Data Rate (Hz)" <- w4213
        n1067 = Reciprocal(x=w4213) -> (1/x=→"Data Period (s)":dbl)
        n1068 = local read "Save ave N"() -> (w4212:dbl)
        n1069 = Divide(x=w4213, y=w4212) -> (x/y=w4211:dbl)
        "Save Data Rate (Hz)" <- w4211
        n1070 = Reciprocal(x=w4211) -> (1/x=→"Save Data Period (s)":dbl)
        n1071 = Multiply(x=w4196, y="# Samples/trap") -> (x*y=w4194:u32)
        "Counts/DMA" <- w4194
        n1072 = property on="Trap Disp. Downsample" class="DigNum (strict)"("Maximum"="# Samples/trap") -> ()  [unwired: 2 in, 2 out]
        n1073 = Multiply(x=w4199, y="# Samples/trap") -> (x*y=w4188:u32)
        "# Samples/channel" <- w4188
        n1074 = Multiply(x=w4188, y=u32 8) -> (x*y=→"Trap AI Elements/DMA read":u32)
        n1075 = local read "APD Int. Count"() -> (w4195:u32)
        n1076 = Multiply(x=w4188, y=u32 3) -> (x*y=→"Trap Pos Elements/DMA read":u32)
        n1077 = Divide(x=w4194, y=w4195) -> (x/y=w4185:dbl)
        "APD Samples/FIFO Acq." <- w4185
        n1078 = Divide(x=w4194, y=40000000.0) -> (x/y=w4192:dbl)
        "DMA Update Period (s)" <- w4192
        n1079 = Multiply(x=2.0, y=w4185) -> (x*y=→"APD Elements/DMA read":dbl)
        n1080 = property on="APD Disp. Downsample" class="DigNum (strict)"("Maximum"=w4185) -> ()  [unwired: 2 in, 2 out]
        n1081 = local read "N sets to save"() -> (w4205:u32)
        n1082 = Multiply(x=w4192, y=w4205) -> (x*y=→"Total Time (s)":dbl)
        "FPGA Averaging" <- FALSE ("FPGA Averaging")
      }
      event "Rescale on Mean": Value Change {
        n1083 = event-data() -> ()  [unwired: 7 out]
        n1084 = And(x=FALSE, y="Rescale on Mean") -> (x .and. y?=w4305:bool)
        n1085 = local write "Rescale on Mean"(w4305) -> ()
        n1086 = local read "Bead Mean (nm)"() -> (w4310:dbl)
        n1087 = Add(x="Amplitude (nm)", y=w4310) -> (x+y=w4308:dbl)
        n1088 = Subtract(x=w4310, y="Amplitude (nm)") -> (x-y=w4307:dbl)
        n1089 = property on="Bead Separation" class="WFChart (strict)"("YScale.Minimum"=w4307) -> ()  [unwired: 2 in, 2 out]
        n1090 = property on="Bead Separation" class="WFChart (strict)"("YScale.Maximum"=w4308) -> ()  [unwired: 2 in, 2 out]
      }
      event "Detector Type": Value Change {
        n1091 = event-data() -> ()  [unwired: 7 out]
        n1092 = local read "AI labels"() -> (w4311:string[])
        n1093 = property on="High Res. Display" class="Ring (strict)"("Strings []"=w4311) -> ()  [unwired: 2 in, 2 out]
        n1094 = Build Array (concatenate)(w4311, "none") -> (w4312:string[])
        n1095 = property on="FFT 1 Choice 1" class="Ring (strict)"("Strings []"=w4312) -> ()  [unwired: 2 in, 2 out]
        n1096 = property on="FFT 1 Choice 2" class="Ring (strict)"("Strings []"=w4312) -> ()  [unwired: 2 in, 2 out]
        n1097 = property on="FFT 2 Choice 1" class="Ring (strict)"("Strings []"=w4312) -> ()  [unwired: 2 in, 2 out]
        n1098 = property on="FFT 2 Choice 2" class="Ring (strict)"("Strings []"=w4312) -> ()  [unwired: 2 in, 2 out]
        n1099 = Bundle("APD 1", "APD 2") -> (w4315:cluster{string, string})  [unwired: 1 out]
        n1100 = Cluster To Array(cluster=w4315) -> (array=w4313:string[])
        n1101 = Build Array (concatenate)(w4313, w4312) -> (w4317:string[])
        n1102 = Array Size(array=w4317) -> (size(s)=w4318:i32)
        n1103 = property on="Signals to Plot" class="LstBox (strict)"("Item Names"=w4317) -> ()  [unwired: 2 in, 2 out]
        n1104 = property on="Signals to Plot" class="LstBox (strict)"("Number of Rows"=w4318) -> ()  [unwired: 2 in, 2 out]
        n1105 = property on="All Signals" class="WFChart (strict)"("LegNumRows"=w4318) -> ()  [unwired: 2 in, 2 out]
      }
      event "Adjust Scale\nto Mean": Value Change {
        n1106 = event-data() -> ()  [unwired: 7 out]
        n1107 = local read "APD 1 Rate (Hz)"() -> (w4327:dbl)
        n1108 = Multiply(x=1000.0, y="Above (kHz)") -> (x*y=w4325:dbl)
        n1109 = Multiply(x=1000.0, y="Below (kHz)") -> (x*y=w4323:dbl)
        n1110 = Add(x=w4325, y=w4327) -> (x+y=w4320:dbl)
        n1111 = Subtract(x=w4327, y=w4323) -> (x-y=w4321:dbl)
        n1112 = property on="APD Chart" class="WFChart (strict)"("YScale.Minimum"=w4321) -> ()  [unwired: 2 in, 2 out]
        n1113 = property on="APD Chart" class="WFChart (strict)"("YScale.Maximum"=w4320) -> ()  [unwired: 2 in, 2 out]
      }
      event "Phase adj. (AI1)", "+ phase (AI1)", "- phase (AI1)": Value Change {
        n1114 = event-data() -> ()  [unwired: 7 out]
        n1115 = Negate(x="Phase adj. (AI1)") -> (-x=w4337:i16)
        n1116 = Select(t=w4337, s="- phase (AI1)", f="Phase adj. (AI1)") -> (s? t:f=w4336:i16)
        n1117 = xnode "Read/Write Control"("FPGA VI Reference In"=w4340, "error in"=w4339, "Phase count adjustment"=w4336) -> ("FPGA VI Reference Out"=w4335:T19, "error out"=w4334:errorcluster)
        n1118 = Or(x="- phase (AI1)", y="+ phase (AI1)") -> (x .or. y?=w4331:bool)
        n1119 = xnode "Read/Write Control"("FPGA VI Reference In"=w4335, "error in"=w4334, "+ phase"=w4331) -> ("error out"=w4330:errorcluster)  [unwired: 1 out]
      }
      event "Signals to Plot": Double Click {
        w4418 = u32 9868950 ("Color Box")
        n1120 = event-data() -> ("Row"=w4420:i32)  [unwired: 9 out]
        n1121 = property on="All Signals" class="WFChart (strict)"("Active Plot"=w4420) -> (error out=w4431:errorcluster)  [unwired: 2 in, 1 out]
        n1122 = property on="All Signals" class="WFChart (strict)" props=["Plot", "Visible?", "Plot", "Plot Color"](error in=w4431) -> (error out=w4430:errorcluster, "Plot.Visible?"=w4429:bool)  [unwired: 1 in, 2 out]
        n1123 = Select(t=FALSE ("Plot.Visible"), s=w4429, f=TRUE ("Plot.Visible")) -> (s? t:f=w4424:bool)
        n1124 = property on="All Signals" class="WFChart (strict)"(error in=w4430, "Plot.Visible?"=w4424) -> (error out=w4426:errorcluster)  [unwired: 1 in, 1 out]
        n1125 = property on="All Signals" class="WFChart (strict)"(error in=w4426) -> (error out=w4421:errorcluster, "Plot.Plot Color"=w4425:u32)  [unwired: 1 in, 1 out]
        n1126 = property on="Signals to Plot" class="LstBox (strict)"(error in=w4421, "Active Row"=w4420) -> (error out=w4419:errorcluster)  [unwired: 1 in, 1 out]
        n1127 = Select(t=w4425, s=w4424, f=u32 0) -> (s? t:f=w4422:u32)
        n1128 = property on="Signals to Plot" class="LstBox (strict)"(error in=w4419, "CellFontColor"=w4422, "SelColor"=w4418, "CellBG"=w4418, "CellFontSize"=u32 20 ("Active Row:Cell Font:Size"), "CellFontBold"=TRUE ("Active Row:Cell Font:Bold")) -> ()  [unwired: 1 in, 2 out]
      }
      event "BD 1 Frequency 1 (MHz)", "BD 1 Frequency 2 (MHz)", "BD 1 Frequency 3 (MHz)", "BD 2 Frequency 1 (MHz)", "BD 2 Frequency 2 (MHz)", "BD 2 Frequency 3 (MHz)", "Trap Delta (MHz)": Value Change {
        # "anytime one of the frequencies is changed, write it to the RF board UNLESS Set 1 is being oscillated. The oscillation\nscript writes the frequencies to the RF board."
        n1129 = event-data() -> ("CtlRef"=w4434:refnum<vi>)  [unwired: 6 out]
        n1130 = control-ref of="Trap Delta (MHz)"() -> (w4433:refnum<vi>)
        n1131 = Equal?(x=w4433, y=w4434) -> (x = y?=w4432:bool)
        n1132 = case shown="False" "Oscillate Set 1" {
          tunnel: w4437 -> [w4457 _]
          tunnel: [w4456 w4460] -> w4436
          tunnel: w4435 -> [w4455 w4460]
          tunnel: w4432 -> [w4440 _]
          frame False {
            n1133 = local read "BD 1 Frequency 2 (MHz)"() -> (w4444:dbl)
            n1134 = local read "BD 1 Frequency 1 (MHz)"() -> (w4442:dbl)
            n1135 = Subtract(x=w4444, y="Trap Delta (MHz)") -> (x-y=w4441:dbl)
            n1136 = Select(t=w4441, s=w4440, f=w4442) -> (s? t:f=w4439:dbl)
            n1137 = local read "Y RF Frequency Limits (MHz)"() -> (w4445:T16)
            n1138 = local read "X RF Frequency Limits (MHz)"() -> (w4446:T16)
            n1139 = local read "BD 1 Frequency 3 (MHz)"() -> (w4458:dbl)
            n1140 = local write "BD 1 Frequency 1 (MHz)"(w4439) -> ()
            n1141 = local read "BD 2 Frequency 1 (MHz)"() -> (w4449:dbl)
            n1142 = local read "BD 2 Frequency 2 (MHz)"() -> (w4448:dbl)
            n1143 = local read "BD 2 Frequency 3 (MHz)"() -> (w4459:dbl)
            n1144 = call "set RF board frequency - interlace.vi"("Board 2 Frequency Limits"=w4445, "Board 1 Frequency Limits"=w4446, "error in"=w4455, "FPGA VI Reference In"=w4457, "Board 2 Frequency 3 (MHz)"=w4459, "Board 1 Frequency 3 (MHz)"=w4458, "Board 2 Frequency 2 (MHz)"=w4448, "Board 2 Frequency 1 (MHz)"=w4449, "Board 1 Frequency 2 (MHz)"=w4444, "Board 1 Frequency 1  (MHz)"=w4439) -> ("error out"=w4456:errorcluster)  [unwired: 1 out]
            n1145 = Subtract(x=w4449, y=w4448) -> (x-y=w4453:dbl)
            n1146 = Subtract(x=w4439, y=w4444) -> (x-y=w4454:dbl)
            n1147 = Square(x=w4453) -> (x^2=w4451:dbl)
            n1148 = Square(x=w4454) -> (x^2=w4452:dbl)
            n1149 = Add(x=w4452, y=w4451) -> (x+y=w4450:dbl)
            n1150 = Square Root(x=w4450) -> (sqrt(x)=w4447:dbl)
            n1151 = local write "Trap Delta (MHz)"(w4447) -> ()
            n1152 = property on="Initial delta (MHz)" class="DigNum (strict)"("Val(Sgnl)"=w4447) -> ()  [unwired: 2 in, 2 out]
          }
          frame True {
          }
        }
      }
      event "Round T1 X": Value Change {
        n1153 = event-data() -> ()  [unwired: 7 out]
        n1154 = local read "BD 1 Frequency 1 (MHz)"() -> (w4463:dbl)
        n1155 = Round To Nearest(number=w4463) -> (nearest integer value=w4462:dbl)
        n1156 = property on="BD 1 Frequency 1 (MHz)" class="DigNum (strict)"("Val(Sgnl)"=w4462) -> ()  [unwired: 2 in, 2 out]
      }
      event "Round T2 X": Value Change {
        n1157 = event-data() -> ()  [unwired: 7 out]
        n1158 = local read "BD 1 Frequency 2 (MHz)"() -> (w4465:dbl)
        n1159 = Round To Nearest(number=w4465) -> (nearest integer value=w4464:dbl)
        n1160 = property on="BD 1 Frequency 2 (MHz)" class="DigNum (strict)"("Val(Sgnl)"=w4464) -> ()  [unwired: 2 in, 2 out]
      }
      event "Stop All": Value Change {
        n1161 = event-data() -> ()  [unwired: 7 out]
        n1162 = local read "Stop All"() -> (w4467:bool)
      }
      event "Delayed Interlace Start": Value Change {
        n1163 = event-data() -> ()  [unwired: 7 out]
        n1164 = flat-sequence {
          frame #0 {
            n1165 = Multiply(x="Delay to Interlace (s)", y=1000.0) -> (x*y=w4470:dbl)
            n1166 = Wait (ms)(milliseconds to wait=w4470) -> ()  [unwired: 1 out]
          }
          frame #1 {
            n1167 = property on="Green laser mode" class="RadioBtnsControl (strict)"("Val(Sgnl)"=enum32{"Laser ON", "Laser OFF", "Interlace"}."Interlace" ("Value (Signaling)")) -> ()  [unwired: 2 in, 2 out]
          }
        }
      }
      event "BD 1 Amplitude 1 (%)", "BD 1 Amplitude 2 (%)", "BD 1 Amplitude 3 (%)", "BD 2 Amplitude 1 (%)", "BD 2 Amplitude 2 (%)", "BD 2 Amplitude 3 (%)", "Trap 1 ON", "Trap 2 ON", "Trap 3 ON", "Feedback On/Off", "All FB On/Off": Value Change {
        w4494 = i16 1 ("f")
        n1168 = event-data() -> ()  [unwired: 7 out]
        n1169 = local write "Trap 1 (ON/OFF)"("Trap 1 ON") -> ()
        n1170 = local write "Trap 2 (ON/OFF)"("Trap 2 ON") -> ()
        n1171 = Boolean To (0,1)(Boolean="Trap 3 ON") -> (0, 1=w4495:i16)
        n1172 = Boolean To (0,1)(Boolean="Trap 1 ON") -> (0, 1=w4496:i16)